vi "Velociprobe_Nanopositioner_Control_RT_2.vi"() -> ()   [LabVIEW 2015] (continued)
      tunnel: [w40 w68 w536 w697 w743 w798 w825 w917] -> w15
      tunnel: [w38 w67 w537 w696 w744 w796 w823 w915] -> w14
      tunnel: w13 -> [w37 w72 w540 w700 w747 w799 w828 w920]
      tunnel: w12 -> [_ w71 w541 w701 w748 w800 w829 w921]
      frame "Initialization", Default {
        w54 = 0  # IRQ Number(s)
        n8 = xnode "Open FPGA VI Reference"("error in"=w37) -> ("FPGA VI Reference Out"=w36:refnum<k20>, "error out"=w49:errorcluster)  [unwired: 1 in]
        n9 = xnode "Invoke Method"("FPGA VI Reference In"=w36, "error in"=w49, "Requested Depth"="Requested Depth") -> ("FPGA VI Reference Out"=w48:refnum<k20>, "error out"=w47:errorcluster, "Actual Depth"=→"Actual Depth":u32)
        n10 = xnode "Read/Write Control"("FPGA VI Reference In"=w48, "error in"=w47, "Datalog Time Period (uSec)"="Datalog Time Period (uSec)", "Datalog Cases"="Datalog Cases", "Interrupt Boolean"=FALSE) -> ("FPGA VI Reference Out"=w46:refnum<k20>, "error out"=w45:errorcluster)
        n11 = xnode "Invoke Method"("FPGA VI Reference In"=w46, "error in"=w45, "IRQ Number(s)"=w54, "Timeout (ms)"="IRQ Timeout (ms)") -> ("FPGA VI Reference Out"=w44:refnum<k20>, "error out"=w43:errorcluster, "Timed Out"=→"IRQ Timed Out":bool, "IRQ(s) Asserted"=w56:i32)
        n12 = xnode "Invoke Method"("FPGA VI Reference In"=w44, "error in"=w43, "IRQ Number(s)"=w56) -> ("FPGA VI Reference Out"=w42:refnum<k20>, "error out"=w41:errorcluster)
        n13 = disable-structure shown="Enabled" {
          disable-tunnel: [w64 errorcluster {"status"=FALSE, "code"=0, "source"=""} ("error out")] -> w50
          frame Disabled {
            n14 = invoke on="Waveform Graph 2" class="WFGraph (strict)" method="Reinit To Default"() -> (error out=w64:errorcluster)  [unwired: 3 in, 2 out]
          }
          frame Enabled {
          }
        }
        n15 = xnode "Read/Write Control"("FPGA VI Reference In"=w42, "error in"=w41) -> ("FPGA VI Reference Out"=w40:refnum<k20>, "error out"=w39:errorcluster, "error out (FPGA)"=w57:errorcluster)
        n16 = Merge Errors "Merge Errors"(w39, w57, w50) -> (w38:errorcluster)
        "Initialization error" <- w38
      }
      frame "Update Controller Info" {
        w296 = dbl[] [1.0, 2.0, 4.0, 5.0]  # Index_soscoeff_zz1
        w135 = dbl[] [1.0, 2.0, 4.0, 5.0]  # Index_soscoeff_yz1
        w156 = dbl[] [1.0, 2.0, 4.0, 5.0]  # Index_soscoeff_xz1
        w187 = dbl[] [1.0, 2.0, 4.0, 5.0]  # Index_soscoeff_zy1
        w317 = dbl[] [1.0, 2.0, 4.0, 5.0]  # Index_soscoeff_yy1
        w208 = dbl[] [1.0, 2.0, 4.0, 5.0]  # Index_soscoeff_xy1
        w234 = dbl[] [1.0, 2.0, 4.0, 5.0]  # Index_soscoeff_zx1
        w343 = dbl[] [1.0, 2.0, 4.0, 5.0]  # Index_soscoeff_xx1
        w260 = dbl[] [1.0, 2.0, 4.0, 5.0]  # Index_soscoeff_yx1
        w116 = "%.10f"  # format (%.3f)
        w124 = "%.10f"  # format (%.3f)
        w137 = "%.10f"  # format (%.3f)
        w145 = "%.10f"  # format (%.3f)
        w168 = "%.10f"  # format (%.3f)
        w176 = "%.10f"  # format (%.3f)
        w189 = "%.10f"  # format (%.3f)
        w197 = "%.10f"  # format (%.3f)
        w215 = "%.10f"  # format (%.3f)
        w223 = "%.10f"  # format (%.3f)
        w241 = "%.10f"  # format (%.3f)
        w249 = "%.10f"  # format (%.3f)
        w277 = "%.10f"  # format (%.3f)
        w285 = "%.10f"  # format (%.3f)
        w298 = "%.10f"  # format (%.3f)
        w306 = "%.10f"  # format (%.3f)
        w107 = fxp<+/-,42,9> 0.0 ("fixed-point type")
        w319 = "%.10f"  # format (%.3f)
        w106 = fxp<+/-,64,9> 0.0 ("fixed-point type")
        w332 = "%.10f"  # format (%.3f)
        w350 = 40000000.0  # FPGA Clock Rate (Hz)
        w83 = 1
        n17 = local read "sos gain SF Controller yy1c"() -> (w271:fxp<+/-,42,9>)
        n18 = local read "sos gain SF Controller yz1c"() -> (w92:fxp<+/-,42,9>)
        n19 = local read "sos gain SF Controller yx1c"() -> (w238:fxp<+/-,42,9>)
        n20 = local read "sos gain SF Controller xy1c"() -> (w161:fxp<+/-,42,9>)
        n21 = local read "sos gain SF Controller zy1c"() -> (w166:fxp<+/-,42,9>)
        n22 = local read "sos gain SF Controller xz1c"() -> (w108:fxp<+/-,42,9>)
        n23 = local read "sos gain SF Controller xx1c"() -> (w321:fxp<+/-,42,9>)
        n24 = local read "sos gain SF Controller zz1c"() -> (w269:fxp<+/-,42,9>)
        n25 = local read "sos gain SF Controller zx1c"() -> (w213:fxp<+/-,42,9>)
        n26 = local read "-a01(2) yy1c"() -> (w275:fxp<+/-,64,9>[])
        n27 = local read "-a02(2) yy1c"() -> (w274:fxp<+/-,64,9>[])
        n28 = local read "-a01(2) yz1c"() -> (w113:fxp<+/-,64,9>[])
        n29 = local read "-a02(2) yz1c"() -> (w114:fxp<+/-,64,9>[])
        n30 = local read "-a01(2) yx1c"() -> (w239:fxp<+/-,64,9>[])
        n31 = local read "-a02(2) yx1c"() -> (w235:fxp<+/-,64,9>[])
        n32 = local read "-a01(2) xy1c"() -> (w157:fxp<+/-,64,9>[])
        n33 = local read "-a02(2) xy1c"() -> (w158:fxp<+/-,64,9>[])
        n34 = local read "-a01(2) zy1c"() -> (w162:fxp<+/-,64,9>[])
        n35 = local read "-a02(2) zy1c"() -> (w163:fxp<+/-,64,9>[])
        n36 = local read "-a01(2) xz1c"() -> (w112:fxp<+/-,64,9>[])
        n37 = local read "-a02(2) xz1c"() -> (w111:fxp<+/-,64,9>[])
        n38 = local read "-a01(2) xx1c"() -> (w330:fxp<+/-,64,9>[])
        n39 = local read "-a02(2) xx1c"() -> (w329:fxp<+/-,64,9>[])
        n40 = local read "-a01(2) zz1c"() -> (w270:fxp<+/-,64,9>[])
        n41 = local read "-a02(2) zz1c"() -> (w266:fxp<+/-,64,9>[])
        n42 = local read "-a01(2) zx1c"() -> (w209:fxp<+/-,64,9>[])
        n43 = local read "-a02(2) zx1c"() -> (w210:fxp<+/-,64,9>[])
        n44 = local read "b01(2) yy1c"() -> (w273:fxp<+/-,64,9>[])
        n45 = local read "b02(2) yy1c"() -> (w272:fxp<+/-,64,9>[])
        n46 = local read "b01(2) yz1c"() -> (w78:fxp<+/-,64,9>[])
        n47 = local read "b02(2) yz1c"() -> (w77:fxp<+/-,64,9>[])
        n48 = local read "b01(2) yx1c"() -> (w236:fxp<+/-,64,9>[])
        n49 = local read "b02(2) yx1c"() -> (w237:fxp<+/-,64,9>[])
        n50 = local read "b01(2) xy1c"() -> (w159:fxp<+/-,64,9>[])
        n51 = local read "b02(2) xy1c"() -> (w160:fxp<+/-,64,9>[])
        n52 = local read "b01(2) zy1c"() -> (w164:fxp<+/-,64,9>[])
        n53 = local read "b02(2) zy1c"() -> (w165:fxp<+/-,64,9>[])
        n54 = local read "b01(2) xz1c"() -> (w110:fxp<+/-,64,9>[])
        n55 = local read "b02(2) xz1c"() -> (w109:fxp<+/-,64,9>[])
        n56 = local read "b01(2) xx1c"() -> (w328:fxp<+/-,64,9>[])
        n57 = local read "b02(2) xx1c"() -> (w327:fxp<+/-,64,9>[])
        n58 = local read "b01(2) zz1c"() -> (w267:fxp<+/-,64,9>[])
        n59 = local read "b02(2) zz1c"() -> (w268:fxp<+/-,64,9>[])
        n60 = local read "b01(2) zx1c"() -> (w211:fxp<+/-,64,9>[])
        n61 = local read "b02(2) zx1c"() -> (w212:fxp<+/-,64,9>[])
        n62 = Or(x="Optics Z Reset", y="Reset All") -> (x .or. y?=w105:bool)
        n63 = Or(x="Sample Z Reset", y="Reset All") -> (x .or. y?=w102:bool)
        n64 = Or(x="Optics X Reset", y="Reset All") -> (x .or. y?=w264:bool)
        n65 = Or(x="Optics Y Reset", y="Reset All") -> (x .or. y?=w262:bool)
        n66 = Or(x="Sample X Reset", y="Reset All") -> (x .or. y?=w104:bool)
        n67 = Or(x="Sample Y Reset", y="Reset All") -> (x .or. y?=w103:bool)
        n68 = call-poly <vilib>:"Read Delimited Spreadsheet.vi"("file path (dialog if empty)"="file path soscoeff_xx1", "format (%.3f)"=w332) -> ("all rows"=w331:dbl[][])  [unwired: 8 in, 5 out]
        n69 = call-poly <vilib>:"Read Delimited Spreadsheet.vi"("file path (dialog if empty)"="file path soscoeff_zy1", "format (%.3f)"=w176) -> ("all rows"=w175:dbl[][])  [unwired: 8 in, 5 out]
        n70 = call-poly <vilib>:"Read Delimited Spreadsheet.vi"("file path (dialog if empty)"="file path soscoeff_xy1", "format (%.3f)"=w197) -> ("all rows"=w196:dbl[][])  [unwired: 8 in, 5 out]
        n71 = call-poly <vilib>:"Read Delimited Spreadsheet.vi"("file path (dialog if empty)"="file path soscoeff_zx1", "format (%.3f)"=w223) -> ("all rows"=w222:dbl[][])  [unwired: 8 in, 5 out]
        n72 = call-poly <vilib>:"Read Delimited Spreadsheet.vi"("file path (dialog if empty)"="file path soscoeff_xz1", "format (%.3f)"=w145) -> ("all rows"=w144:dbl[][])  [unwired: 8 in, 5 out]
        n73 = call-poly <vilib>:"Read Delimited Spreadsheet.vi"("file path (dialog if empty)"="file path soscoeff_yx1", "format (%.3f)"=w249) -> ("all rows"=w248:dbl[][])  [unwired: 8 in, 5 out]
        n74 = call-poly <vilib>:"Read Delimited Spreadsheet.vi"("file path (dialog if empty)"="file path soscoeff_yy1", "format (%.3f)"=w306) -> ("all rows"=w305:dbl[][])  [unwired: 8 in, 5 out]
        n75 = call-poly <vilib>:"Read Delimited Spreadsheet.vi"("file path (dialog if empty)"="file path soscoeff_yz1", "format (%.3f)"=w124) -> ("all rows"=w123:dbl[][])  [unwired: 8 in, 5 out]
        n76 = call-poly <vilib>:"Read Delimited Spreadsheet.vi"("file path (dialog if empty)"="file path soscoeff_zz1", "format (%.3f)"=w285) -> ("all rows"=w284:dbl[][])  [unwired: 8 in, 5 out]
        n77 = Transpose 2D Array(2D array=w331) -> (transposed array=w342:dbl[][])
        n78 = Transpose 2D Array(2D array=w175) -> (transposed array=w186:dbl[][])
        n79 = Transpose 2D Array(2D array=w196) -> (transposed array=w207:dbl[][])
        n80 = Transpose 2D Array(2D array=w222) -> (transposed array=w233:dbl[][])
        n81 = Transpose 2D Array(2D array=w144) -> (transposed array=w155:dbl[][])
        n82 = Transpose 2D Array(2D array=w248) -> (transposed array=w259:dbl[][])
        n83 = Transpose 2D Array(2D array=w305) -> (transposed array=w316:dbl[][])
        n84 = Transpose 2D Array(2D array=w123) -> (transposed array=w134:dbl[][])
        n85 = Transpose 2D Array(2D array=w284) -> (transposed array=w295:dbl[][])
        n86 = call-poly <vilib>:"Read Delimited Spreadsheet.vi"("file path (dialog if empty)"="file path sos gain SF Controller_xx1", "format (%.3f)"=w319) -> ("all rows"=w318:dbl[][])  [unwired: 8 in, 5 out]
        n87 = call-poly <vilib>:"Read Delimited Spreadsheet.vi"("file path (dialog if empty)"="file path sos gain SF Controller_zy1", "format (%.3f)"=w168) -> ("all rows"=w167:dbl[][])  [unwired: 8 in, 5 out]
        n88 = call-poly <vilib>:"Read Delimited Spreadsheet.vi"("file path (dialog if empty)"="file path sos gain SF Controller_xy1", "format (%.3f)"=w189) -> ("all rows"=w188:dbl[][])  [unwired: 8 in, 5 out]
        n89 = call-poly <vilib>:"Read Delimited Spreadsheet.vi"("file path (dialog if empty)"="file path sos gain SF Controller_zx1", "format (%.3f)"=w215) -> ("all rows"=w214:dbl[][])  [unwired: 8 in, 5 out]
        n90 = call-poly <vilib>:"Read Delimited Spreadsheet.vi"("file path (dialog if empty)"="file path sos gain SF Controller_xz1", "format (%.3f)"=w137) -> ("all rows"=w136:dbl[][])  [unwired: 8 in, 5 out]
        n91 = call-poly <vilib>:"Read Delimited Spreadsheet.vi"("file path (dialog if empty)"="file path sos gain SF Controller_yx1", "format (%.3f)"=w241) -> ("all rows"=w240:dbl[][])  [unwired: 8 in, 5 out]
        n92 = call-poly <vilib>:"Read Delimited Spreadsheet.vi"("file path (dialog if empty)"="file path sos gain SF Controller_yy1", "format (%.3f)"=w298) -> ("all rows"=w297:dbl[][])  [unwired: 8 in, 5 out]
        n93 = call-poly <vilib>:"Read Delimited Spreadsheet.vi"("file path (dialog if empty)"="file path sos gain SF Controller_yz1", "format (%.3f)"=w116) -> ("all rows"=w115:dbl[][])  [unwired: 8 in, 5 out]
        n94 = call-poly <vilib>:"Read Delimited Spreadsheet.vi"("file path (dialog if empty)"="file path sos gain SF Controller_zz1", "format (%.3f)"=w277) -> ("all rows"=w276:dbl[][])  [unwired: 8 in, 5 out]
        n95 = xnode "Read/Write Control"("FPGA VI Reference In"=w71, "error in"=w72, "Controller Time Period (uSec)"="Controller Time Period (uSec)", "Controller Output Time Period (uSec)"="Controller Output Time Period (uSec)", "System Loop Type"="System Loop Type", "Controller Output Upper Limit"="Controller Output Upper Limit", "Controller Output Lower Limit"="Controller Output Lower Limit", "X-Stage nm to V Scaling"="X-Stage nm to V Scaling", "X-Stage Scaling Direction"="X-Stage Scaling Direction", "Y-Stage nm to V Scaling"="Y-Stage nm to V Scaling", "Z-Stage nm to V Scaling"="Z-Stage nm to V Scaling", "Plant Output Time Period (uSec)"="Plant Output Time Period (uSec)", "Reset Optics X"=w264, "Reset Optics Y"=w262, "Reset Optics Z"=w105, "Reset Sample X"=w104, "Reset Sample Y"=w103, "Reset Sample Z"=w102, "Optics X Stage Resolution (nm)"="Optics X Stage Resolution (nm)", "Optics Y Stage Resolution (nm)"="Optics Y Stage Resolution (nm)", "Optics Z Stage Resolution (nm)"="Optics Z Stage Resolution (nm)", "Sample X Stage Resolution (nm)"="Sample X Stage Resolution (nm)", "Sample Y Stage Resolution (nm)"="Sample Y Stage Resolution (nm)", "Sample Z Stage Resolution (nm)"="Sample Z Stage Resolution (nm)", "Scaling mV to V"="Scaling mV to V", "-a01(2) xx1"=w330, "-a02(2) xx1"=w329, "b01(2) xx1"=w328, "b02(2) xx1"=w327, "sos gain SF Controller xx1"=w321, "-a01(2) yy1"=w275, "-a02(2) yy1"=w274, "b01(2) yy1"=w273, "b02(2) yy1"=w272, "sos gain SF Controller yy1"=w271, "-a01(2) zz1"=w270, "-a02(2) zz1"=w266, "b01(2) zz1"=w267, "b02(2) zz1"=w268, "sos gain SF Controller zz1"=w269, "-a01(2) yx1"=w239, "-a02(2) yx1"=w235, "b01(2) yx1"=w236, "b02(2) yx1"=w237, "sos gain SF Controller yx1"=w238, "-a01(2) zx1"=w209, "-a02(2) zx1"=w210, "b01(2) zx1"=w211, "b02(2) zx1"=w212, "sos gain SF Controller zx1"=w213, "-a01(2) xy1"=w157, "-a02(2) xy1"=w158, "b01(2) xy1"=w159, "b02(2) xy1"=w160, "sos gain SF Controller xy1"=w161, "-a01(2) zy1"=w162, "-a02(2) zy1"=w163, "b01(2) zy1"=w164, "b02(2) zy1"=w165, "sos gain SF Controller zy1"=w166, "-a01(2) xz1"=w112, "-a02(2) xz1"=w111, "b01(2) xz1"=w110, "b02(2) xz1"=w109, "sos gain SF Controller xz1"=w108, "-a01(2) yz1"=w113, "-a02(2) yz1"=w114, "b01(2) yz1"=w78, "b02(2) yz1"=w77, "sos gain SF Controller yz1"=w92, "Analog Input Time Period (uSec)"="Analog Input Time Period (uSec)", "Optics and or Sample Stage"="Optics and or Sample Stage", "Y-Stage Scaling Direction"="Y-Stage Scaling Direction", "Z-Stage Scaling Direction"="Z-Stage Scaling Direction") -> ("FPGA VI Reference Out"=w70:refnum<k20>, "error out"=w69:errorcluster)
        n96 = for {
          tunnel: w343 -> [w519] mode=indexing
          tunnel: w342 -> [w518]
          tunnel: [w517] -> _ mode=indexing
          shift-right: [w517] -> w334
          shift-left: _ -> [w516]
          shift-left: _ -> [w515]
          shift-left: _ -> [w514]
          tunnel: [w516] -> w335
          tunnel: [w515] -> w336
          tunnel: [w514] -> w337
          n97 = Index Array "Index Array"(array=w518, index (row)=w519) -> (element=w517:dbl[])  [unwired: 1 in]
        }
        n98 = Index Array(array=w318, index (row)=0 ("index (row) 6")) -> (element=w326:dbl[])  [unwired: 1 in]
        n99 = for {
          tunnel: w187 -> [w417] mode=indexing
          tunnel: w186 -> [w416]
          tunnel: [w415] -> _ mode=indexing
          shift-right: [w415] -> w178
          shift-left: _ -> [w414]
          shift-left: _ -> [w413]
          shift-left: _ -> [w412]
          tunnel: [w414] -> w179
          tunnel: [w413] -> w180
          tunnel: [w412] -> w181
          n100 = Index Array "Index Array"(array=w416, index (row)=w417) -> (element=w415:dbl[])  [unwired: 1 in]
        }
        n101 = Index Array(array=w167, index (row)=0 ("index (row) 18")) -> (element=w174:dbl[])  [unwired: 1 in]
        n102 = for {
          tunnel: w208 -> [w434] mode=indexing
          tunnel: w207 -> [w433]
          tunnel: [w432] -> _ mode=indexing
          shift-right: [w432] -> w199
          shift-left: _ -> [w431]
          shift-left: _ -> [w430]
          shift-left: _ -> [w429]
          tunnel: [w431] -> w200
          tunnel: [w430] -> w201
          tunnel: [w429] -> w202
          n103 = Index Array "Index Array"(array=w433, index (row)=w434) -> (element=w432:dbl[])  [unwired: 1 in]
        }
        n104 = Index Array(array=w188, index (row)=0 ("index (row) 16")) -> (element=w195:dbl[])  [unwired: 1 in]
        n105 = for {
          tunnel: w234 -> [w451] mode=indexing
          tunnel: w233 -> [w450]
          tunnel: [w449] -> _ mode=indexing
          shift-right: [w449] -> w225
          shift-left: _ -> [w448]
          shift-left: _ -> [w447]
          shift-left: _ -> [w446]
          tunnel: [w448] -> w226
          tunnel: [w447] -> w227
          tunnel: [w446] -> w228
          n106 = Index Array "Index Array"(array=w450, index (row)=w451) -> (element=w449:dbl[])  [unwired: 1 in]
        }
        n107 = Index Array(array=w214, index (row)=0 ("index (row) 14")) -> (element=w221:dbl[])  [unwired: 1 in]
        n108 = for {
          tunnel: w156 -> [w400] mode=indexing
          tunnel: w155 -> [w399]
          tunnel: [w398] -> _ mode=indexing
          shift-right: [w398] -> w147
          shift-left: _ -> [w397]
          shift-left: _ -> [w396]
          shift-left: _ -> [w395]
          tunnel: [w397] -> w148
          tunnel: [w396] -> w149
          tunnel: [w395] -> w150
          n109 = Index Array "Index Array"(array=w399, index (row)=w400) -> (element=w398:dbl[])  [unwired: 1 in]
        }
        n110 = Index Array(array=w136, index (row)=0 ("index (row) 20")) -> (element=w143:dbl[])  [unwired: 1 in]
        n111 = for {
          tunnel: w260 -> [w468] mode=indexing
          tunnel: w259 -> [w467]
          tunnel: [w466] -> _ mode=indexing
          shift-right: [w466] -> w251
          shift-left: _ -> [w465]
          shift-left: _ -> [w464]
          shift-left: _ -> [w463]
          tunnel: [w465] -> w252
          tunnel: [w464] -> w253
          tunnel: [w463] -> w254
          n112 = Index Array "Index Array"(array=w467, index (row)=w468) -> (element=w466:dbl[])  [unwired: 1 in]
        }
        n113 = Index Array(array=w240, index (row)=0 ("index (row) 12")) -> (element=w247:dbl[])  [unwired: 1 in]
        n114 = for {
          tunnel: w317 -> [w502] mode=indexing
          tunnel: w316 -> [w501]
          tunnel: [w500] -> _ mode=indexing
          shift-right: [w500] -> w308
          shift-left: _ -> [w499]
          shift-left: _ -> [w498]
          shift-left: _ -> [w497]
          tunnel: [w499] -> w309
          tunnel: [w498] -> w310
          tunnel: [w497] -> w311
          n115 = Index Array "Index Array"(array=w501, index (row)=w502) -> (element=w500:dbl[])  [unwired: 1 in]
        }
        n116 = Index Array(array=w297, index (row)=0 ("index (row) 8")) -> (element=w304:dbl[])  [unwired: 1 in]
        n117 = for {
          tunnel: w135 -> [w383] mode=indexing
          tunnel: w134 -> [w382]
          tunnel: [w381] -> _ mode=indexing
          shift-right: [w381] -> w126
          shift-left: _ -> [w380]
          shift-left: _ -> [w379]
          shift-left: _ -> [w378]
          tunnel: [w380] -> w127
          tunnel: [w379] -> w128
          tunnel: [w378] -> w129
          n118 = Index Array "Index Array"(array=w382, index (row)=w383) -> (element=w381:dbl[])  [unwired: 1 in]
        }
        n119 = Index Array(array=w115, index (row)=0 ("index (row) 22")) -> (element=w122:dbl[])  [unwired: 1 in]
        n120 = Index Array(array=w276, index (row)=0 ("index (row) 10")) -> (element=w283:dbl[])  [unwired: 1 in]
        n121 = for {
          tunnel: w296 -> [w485] mode=indexing
          tunnel: w295 -> [w484]
          tunnel: [w483] -> _ mode=indexing
          shift-right: [w483] -> w287
          shift-left: _ -> [w482]
          shift-left: _ -> [w481]
          shift-left: _ -> [w480]
          tunnel: [w482] -> w288
          tunnel: [w481] -> w289
          tunnel: [w480] -> w290
          n122 = Index Array "Index Array"(array=w484, index (row)=w485) -> (element=w483:dbl[])  [unwired: 1 in]
        }
        n123 = Index Array(array=w326, index=0 ("index (row) 7")) -> (element=w324:dbl)
        n124 = Index Array(array=w174, index=0 ("index (row) 19")) -> (element=w172:dbl)
        n125 = Index Array(array=w195, index=0 ("index (row) 17")) -> (element=w193:dbl)
        n126 = Index Array(array=w221, index=0 ("index (row) 15")) -> (element=w219:dbl)
        n127 = Index Array(array=w143, index=0 ("index (row) 21")) -> (element=w141:dbl)
        n128 = Index Array(array=w247, index=0 ("index (row) 13")) -> (element=w245:dbl)
        n129 = Index Array(array=w304, index=0 ("index (row) 9")) -> (element=w302:dbl)
        n130 = Index Array(array=w122, index=0 ("index (row) 23")) -> (element=w120:dbl)
        n131 = Index Array(array=w283, index=0 ("index (row) 11")) -> (element=w281:dbl)
        n132 = xnode "Read/Write Control"("FPGA VI Reference In"=w70, "error in"=w69) -> ("FPGA VI Reference Out"=w68:refnum<k20>, "error out"=w67:errorcluster, "PI X-Stage Input (V)"=→"PI X-Stage Input (V)":fxp<+/-,20,5>, "PI Y-Stage Input (V)"=→"PI Y-Stage Input (V)":fxp<+/-,20,5>, "PI Z-Stage Input (V)"=→"PI Z-Stage Input (V)":fxp<+/-,20,5>, "X-Stage Input In Range?"=→"X-Stage Input In Range?":bool, "Y-Stage Input In Range?"=→"Y-Stage Input In Range?":bool, "Z-Stage Input In Range?"=→"Z-Stage Input In Range?":bool, "Measured Controller Time Period (Ticks)"=w351:u32, "Measured Controller Output Time Period (Ticks)"=w348:u32, "Measured Plant Output Time Period (Ticks)"=w84:u32, "Measured Analog Input Time Period (Ticks)"=→"Measured Analog Input Time Period (Ticks)":u32)
        "Measured Controller Time Period (Ticks)" <- w351
        "Measured Controller Output Time Period (Ticks)" <- w348
        "Measured Plant Output Time Period (Ticks)" <- w84
        n133 = To Fixed-Point(fixed-point type=w107, number=w193) -> (fixed-point=→"sos gain SF Controller xy1c":fxp<+/-,42,9>)
        n134 = To Fixed-Point(fixed-point type=w107, number=w302) -> (fixed-point=→"sos gain SF Controller yy1c":fxp<+/-,42,9>)
        n135 = To Fixed-Point(fixed-point type=w107, number=w172) -> (fixed-point=→"sos gain SF Controller zy1c":fxp<+/-,42,9>)
        n136 = To Fixed-Point(fixed-point type=w107, number=w141) -> (fixed-point=→"sos gain SF Controller xz1c":fxp<+/-,42,9>)
        n137 = To Fixed-Point(fixed-point type=w107, number=w120) -> (fixed-point=→"sos gain SF Controller yz1c":fxp<+/-,42,9>)
        n138 = To Fixed-Point(fixed-point type=w107, number=w245) -> (fixed-point=→"sos gain SF Controller yx1c":fxp<+/-,42,9>)
        n139 = To Fixed-Point(fixed-point type=w107, number=w219) -> (fixed-point=→"sos gain SF Controller zx1c":fxp<+/-,42,9>)
        n140 = To Fixed-Point(fixed-point type=w107, number=w281) -> (fixed-point=→"sos gain SF Controller zz1c":fxp<+/-,42,9>)
        n141 = To Fixed-Point(fixed-point type=w107, number=w324) -> (fixed-point=→"sos gain SF Controller xx1c":fxp<+/-,42,9>)
        n142 = Divide(x=w83, y=w350) -> (x/y=w85:dbl)
        n143 = Multiply(x=w85, y=w351) -> (x*y=w352:dbl)
        "Measured Controller Loop Rate (secs)" <- w352
        n144 = Multiply(x=w85, y=w348) -> (x*y=w360:dbl)
        "Measured Controller Output Loop Rate (secs)" <- w360
        n145 = Multiply(x=w85, y=w84) -> (x*y=w356:dbl)
        "Measured Plant Output Loop Rate (secs)" <- w356
        n146 = Multiply(x=w85, y=w84) -> (x*y=w89:dbl)
        "Measured Analog Input Loop Rate (secs)" <- w89
        n147 = for {
          tunnel: w179 -> [w428] mode=indexing
          tunnel: [w427] -> w185 mode=indexing
          tunnel: w178 -> [w426] mode=indexing
          tunnel: w181 -> [w425] mode=indexing
          tunnel: w180 -> [w424] mode=indexing
          tunnel: [w423] -> w184 mode=indexing
          tunnel: [w422] -> w183 mode=indexing
          tunnel: [w421] -> w182 mode=indexing
          tunnel: w106 -> [w418]
          n148 = Negate(x=w428) -> (-x=w420:dbl)
          n149 = Negate(x=w426) -> (-x=w419:dbl)
          n150 = To Fixed-Point(fixed-point type=w418, number=w420) -> (fixed-point=w427:fxp<+/-,64,9>)
          n151 = To Fixed-Point(fixed-point type=w418, number=w419) -> (fixed-point=w423:fxp<+/-,64,9>)
          n152 = To Fixed-Point(fixed-point type=w418, number=w425) -> (fixed-point=w422:fxp<+/-,64,9>)
          n153 = To Fixed-Point(fixed-point type=w418, number=w424) -> (fixed-point=w421:fxp<+/-,64,9>)
        }
        "-a01(2) zy1c" <- w185
        "-a02(2) zy1c" <- w184
        "b01(2) zy1c" <- w183
        "b02(2) zy1c" <- w182
        n154 = for {
          tunnel: w335 -> [w530] mode=indexing
          tunnel: [w529] -> w341 mode=indexing
          tunnel: w334 -> [w528] mode=indexing
          tunnel: w337 -> [w527] mode=indexing
          tunnel: w336 -> [w526] mode=indexing
          tunnel: [w525] -> w340 mode=indexing
          tunnel: [w524] -> w339 mode=indexing
          tunnel: [w523] -> w338 mode=indexing
          tunnel: w106 -> [w520]
          n155 = Negate(x=w530) -> (-x=w522:dbl)
          n156 = Negate(x=w528) -> (-x=w521:dbl)
          n157 = To Fixed-Point(fixed-point type=w520, number=w522) -> (fixed-point=w529:fxp<+/-,64,9>)
          n158 = To Fixed-Point(fixed-point type=w520, number=w521) -> (fixed-point=w525:fxp<+/-,64,9>)
          n159 = To Fixed-Point(fixed-point type=w520, number=w527) -> (fixed-point=w524:fxp<+/-,64,9>)
          n160 = To Fixed-Point(fixed-point type=w520, number=w526) -> (fixed-point=w523:fxp<+/-,64,9>)
        }
        "-a01(2) xx1c" <- w341
        "-a02(2) xx1c" <- w340
        "b01(2) xx1c" <- w339
        "b02(2) xx1c" <- w338
        n161 = for {
          tunnel: w200 -> [w445] mode=indexing
          tunnel: [w444] -> w206 mode=indexing
          tunnel: w199 -> [w443] mode=indexing
          tunnel: w202 -> [w442] mode=indexing
          tunnel: w201 -> [w441] mode=indexing
          tunnel: [w440] -> w205 mode=indexing
          tunnel: [w439] -> w204 mode=indexing
          tunnel: [w438] -> w203 mode=indexing
          tunnel: w106 -> [w435]
          n162 = Negate(x=w445) -> (-x=w437:dbl)
          n163 = Negate(x=w443) -> (-x=w436:dbl)
          n164 = To Fixed-Point(fixed-point type=w435, number=w437) -> (fixed-point=w444:fxp<+/-,64,9>)
          n165 = To Fixed-Point(fixed-point type=w435, number=w436) -> (fixed-point=w440:fxp<+/-,64,9>)
          n166 = To Fixed-Point(fixed-point type=w435, number=w442) -> (fixed-point=w439:fxp<+/-,64,9>)
          n167 = To Fixed-Point(fixed-point type=w435, number=w441) -> (fixed-point=w438:fxp<+/-,64,9>)
        }
        "-a01(2) xy1c" <- w206
        "-a02(2) xy1c" <- w205
        "b01(2) xy1c" <- w204
        "b02(2) xy1c" <- w203
        n168 = for {
          tunnel: w148 -> [w411] mode=indexing
          tunnel: [w410] -> w154 mode=indexing
          tunnel: w147 -> [w409] mode=indexing
          tunnel: w150 -> [w408] mode=indexing
          tunnel: w149 -> [w407] mode=indexing
          tunnel: [w406] -> w153 mode=indexing
          tunnel: [w405] -> w152 mode=indexing
          tunnel: [w404] -> w151 mode=indexing
          tunnel: w106 -> [w401]
          n169 = Negate(x=w411) -> (-x=w403:dbl)
          n170 = Negate(x=w409) -> (-x=w402:dbl)
          n171 = To Fixed-Point(fixed-point type=w401, number=w403) -> (fixed-point=w410:fxp<+/-,64,9>)
          n172 = To Fixed-Point(fixed-point type=w401, number=w402) -> (fixed-point=w406:fxp<+/-,64,9>)
          n173 = To Fixed-Point(fixed-point type=w401, number=w408) -> (fixed-point=w405:fxp<+/-,64,9>)
          n174 = To Fixed-Point(fixed-point type=w401, number=w407) -> (fixed-point=w404:fxp<+/-,64,9>)
        }
        "-a01(2) xz1c" <- w154
        "-a02(2) xz1c" <- w153
        "b01(2) xz1c" <- w152
        "b02(2) xz1c" <- w151
        n175 = for {
          tunnel: w309 -> [w513] mode=indexing
          tunnel: [w512] -> w315 mode=indexing
          tunnel: w308 -> [w511] mode=indexing
          tunnel: w311 -> [w510] mode=indexing
          tunnel: w310 -> [w509] mode=indexing
          tunnel: [w508] -> w314 mode=indexing
          tunnel: [w507] -> w313 mode=indexing
          tunnel: [w506] -> w312 mode=indexing
          tunnel: w106 -> [w503]
          n176 = Negate(x=w513) -> (-x=w505:dbl)
          n177 = Negate(x=w511) -> (-x=w504:dbl)
          n178 = To Fixed-Point(fixed-point type=w503, number=w505) -> (fixed-point=w512:fxp<+/-,64,9>)
          n179 = To Fixed-Point(fixed-point type=w503, number=w504) -> (fixed-point=w508:fxp<+/-,64,9>)
          n180 = To Fixed-Point(fixed-point type=w503, number=w510) -> (fixed-point=w507:fxp<+/-,64,9>)
          n181 = To Fixed-Point(fixed-point type=w503, number=w509) -> (fixed-point=w506:fxp<+/-,64,9>)
        }
        "-a01(2) yy1c" <- w315
        "-a02(2) yy1c" <- w314
        "b01(2) yy1c" <- w313
        "b02(2) yy1c" <- w312
        n182 = for {
          tunnel: w226 -> [w462] mode=indexing
          tunnel: [w461] -> w232 mode=indexing
          tunnel: w225 -> [w460] mode=indexing
          tunnel: w228 -> [w459] mode=indexing
          tunnel: w227 -> [w458] mode=indexing
          tunnel: [w457] -> w231 mode=indexing
          tunnel: [w456] -> w230 mode=indexing
          tunnel: [w455] -> w229 mode=indexing
          tunnel: w106 -> [w452]
          n183 = Negate(x=w462) -> (-x=w454:dbl)
          n184 = Negate(x=w460) -> (-x=w453:dbl)
          n185 = To Fixed-Point(fixed-point type=w452, number=w454) -> (fixed-point=w461:fxp<+/-,64,9>)
          n186 = To Fixed-Point(fixed-point type=w452, number=w453) -> (fixed-point=w457:fxp<+/-,64,9>)
          n187 = To Fixed-Point(fixed-point type=w452, number=w459) -> (fixed-point=w456:fxp<+/-,64,9>)
          n188 = To Fixed-Point(fixed-point type=w452, number=w458) -> (fixed-point=w455:fxp<+/-,64,9>)
        }
        "-a01(2) zx1c" <- w232
        "-a02(2) zx1c" <- w231
        "b01(2) zx1c" <- w230
        "b02(2) zx1c" <- w229
        n189 = for {
          tunnel: w252 -> [w479] mode=indexing
          tunnel: [w478] -> w258 mode=indexing
          tunnel: w251 -> [w477] mode=indexing
          tunnel: w254 -> [w476] mode=indexing
          tunnel: w253 -> [w475] mode=indexing
          tunnel: [w474] -> w257 mode=indexing
          tunnel: [w473] -> w256 mode=indexing
          tunnel: [w472] -> w255 mode=indexing
          tunnel: w106 -> [w469]
          n190 = Negate(x=w479) -> (-x=w471:dbl)
          n191 = Negate(x=w477) -> (-x=w470:dbl)
          n192 = To Fixed-Point(fixed-point type=w469, number=w471) -> (fixed-point=w478:fxp<+/-,64,9>)
          n193 = To Fixed-Point(fixed-point type=w469, number=w470) -> (fixed-point=w474:fxp<+/-,64,9>)
          n194 = To Fixed-Point(fixed-point type=w469, number=w476) -> (fixed-point=w473:fxp<+/-,64,9>)
          n195 = To Fixed-Point(fixed-point type=w469, number=w475) -> (fixed-point=w472:fxp<+/-,64,9>)
        }
        "-a01(2) yx1c" <- w258
        "-a02(2) yx1c" <- w257
        "b01(2) yx1c" <- w256
        "b02(2) yx1c" <- w255
        n196 = for {
          tunnel: w127 -> [w394] mode=indexing
          tunnel: [w393] -> w133 mode=indexing
          tunnel: w126 -> [w392] mode=indexing
          tunnel: w129 -> [w391] mode=indexing
          tunnel: w128 -> [w390] mode=indexing
          tunnel: [w389] -> w132 mode=indexing
          tunnel: [w388] -> w131 mode=indexing
          tunnel: [w387] -> w130 mode=indexing
          tunnel: w106 -> [w384]
          n197 = Negate(x=w394) -> (-x=w386:dbl)
          n198 = Negate(x=w392) -> (-x=w385:dbl)
          n199 = To Fixed-Point(fixed-point type=w384, number=w386) -> (fixed-point=w393:fxp<+/-,64,9>)
          n200 = To Fixed-Point(fixed-point type=w384, number=w385) -> (fixed-point=w389:fxp<+/-,64,9>)
          n201 = To Fixed-Point(fixed-point type=w384, number=w391) -> (fixed-point=w388:fxp<+/-,64,9>)
          n202 = To Fixed-Point(fixed-point type=w384, number=w390) -> (fixed-point=w387:fxp<+/-,64,9>)
        }
        "-a01(2) yz1c" <- w133
        "-a02(2) yz1c" <- w132
        "b01(2) yz1c" <- w131
        "b02(2) yz1c" <- w130
        n203 = Divide(x=w83, y=w352) -> (x/y=w363:dbl)
        n204 = Divide(x=w83, y=w360) -> (x/y=w359:dbl)
        n205 = Divide(x=w83, y=w356) -> (x/y=w355:dbl)
        n206 = for {
          tunnel: w288 -> [w496] mode=indexing
          tunnel: [w495] -> w294 mode=indexing
          tunnel: w287 -> [w494] mode=indexing
          tunnel: w290 -> [w493] mode=indexing
          tunnel: w289 -> [w492] mode=indexing
          tunnel: [w491] -> w293 mode=indexing
          tunnel: [w490] -> w292 mode=indexing
          tunnel: [w489] -> w291 mode=indexing
          tunnel: w106 -> [w486]
          n207 = Negate(x=w496) -> (-x=w488:dbl)
          n208 = Negate(x=w494) -> (-x=w487:dbl)
          n209 = To Fixed-Point(fixed-point type=w486, number=w488) -> (fixed-point=w495:fxp<+/-,64,9>)
          n210 = To Fixed-Point(fixed-point type=w486, number=w487) -> (fixed-point=w491:fxp<+/-,64,9>)
          n211 = To Fixed-Point(fixed-point type=w486, number=w493) -> (fixed-point=w490:fxp<+/-,64,9>)
          n212 = To Fixed-Point(fixed-point type=w486, number=w492) -> (fixed-point=w489:fxp<+/-,64,9>)
        }
        "-a01(2) zz1c" <- w294
        "-a02(2) zz1c" <- w293
        "b01(2) zz1c" <- w292
        "b02(2) zz1c" <- w291
        n213 = Divide(x=w83, y=w89) -> (x/y=w88:dbl)
        n214 = Divide(x=w363, y=1000) -> (x/y=→"Measured Controller Loop Rate (kHz)":dbl)
        n215 = Divide(x=w359, y=1000) -> (x/y=→"Measured Controller Output Loop Rate (kHz)":dbl)
        n216 = Divide(x=w355, y=1000) -> (x/y=→"Measured Plant Output Loop Rate (kHz)":dbl)
        n217 = Divide(x=w88, y=1000) -> (x/y=→"Measured Analog Input Loop Rate (kHz)":dbl)
      }
      frame "Update Reference Info" {
        w608 = 40000000.0  # FPGA Clock Rate (Hz)
        w602 = 1
        w615 = 40000000.0  # FPGA Clock Rate (Hz)
        w609 = 1
        w620 = errorcluster {"status"=FALSE, "code"=0, "source"=""}  # error in (no error)
        w623 = errorcluster {"status"=FALSE, "code"=0, "source"=""}  # error in (no error)
        w637 = 40000000.0  # FPGA Clock Rate (Hz)
        w631 = 1
        w649 = errorcluster {"status"=FALSE, "code"=0, "source"=""}  # error in (no error)
        w616 = 40000000.0  # FPGA clock rate (Hz)
        n218 = case shown="\"EPICS Snake Scan\"" "Snake Scan Reference FPGA or EPICS" {
          tunnel: ["X Ramp Start (nm)" w667] -> w549
          tunnel: ["X Ramp End (nm)" w666] -> w548
          tunnel: ["Fly Scan Start" w672] -> w547
          tunnel: ["Y Ramp Start (nm)" w665] -> w546
          tunnel: ["Y Ramp End (nm)" w664] -> w545
          tunnel: ["Y Step Size (nm)" w668] -> w544
          tunnel: ["X Step Size (nm)" w671] -> w543
          tunnel: [w658 w669] -> w542
          tunnel: ["Y Step Size (nm)" w668] -> w535
          tunnel: ["X Ramp Start (nm)" w667] -> w534
          tunnel: ["X Ramp End (nm)" w666] -> w533
          tunnel: ["Y Ramp Start (nm)" w665] -> w532
          tunnel: ["Y Ramp End (nm)" w664] -> w531
          frame "FPGA Snake Scan", Default {
            n219 = local read "DT Frequency (Hz)"() -> (w658:dbl)
          }
          frame "EPICS Snake Scan" {
            w670 = fxp<+/-,16,16> 0.0 ("fixed-point type")
            n220 = shared-variable "RT CompactRIO Target\\RT_EPICS_Shared_Variables.lvlib\\2iddVELO:VP:Trigger_Freq_Hz"() -> (w669:dbl)  [unwired: 1 in, 1 out]
            "2iddVELO:VP:Trigger_Freq_Hz" <- w669
            n221 = shared-variable "RT CompactRIO Target\\RT_EPICS_Shared_Variables.lvlib\\2iddVELO:VP:Y_Step_Size_nm"() -> (w674:dbl)  [unwired: 1 in, 1 out]
            "2iddVELO:VP:Y_Step_Size_nm" <- w674
            n222 = shared-variable "RT CompactRIO Target\\RT_EPICS_Shared_Variables.lvlib\\2iddVELO:VP:X_Step_Size_nm"() -> (w673:dbl)  [unwired: 1 in, 1 out]
            "2iddVELO:VP:X_Step_Size_nm" <- w673
            n223 = shared-variable "RT CompactRIO Target\\RT_EPICS_Shared_Variables.lvlib\\2iddVELO:VP:Y_Start_nm"() -> (w675:dbl)  [unwired: 1 in, 1 out]
            n224 = shared-variable "RT CompactRIO Target\\RT_EPICS_Shared_Variables.lvlib\\2iddVELO:VP:Y_End_nm"() -> (w663:dbl)  [unwired: 1 in, 1 out]
            n225 = shared-variable "RT CompactRIO Target\\RT_EPICS_Shared_Variables.lvlib\\2iddVELO:VP:Flyscan_Start"() -> (w672:bool)  [unwired: 1 in, 1 out]
            "2iddVELO:VP:Flyscan_Start" <- w672
            n226 = shared-variable "RT CompactRIO Target\\RT_EPICS_Shared_Variables.lvlib\\2iddVELO:VP:X_Start_nm"() -> (w677:dbl)  [unwired: 1 in, 1 out]
            "2iddVELO:VP:X_Start_nm" <- w677
            n227 = shared-variable "RT CompactRIO Target\\RT_EPICS_Shared_Variables.lvlib\\2iddVELO:VP:X_End_nm"() -> (w676:dbl)  [unwired: 1 in, 1 out]
            "2iddVELO:VP:X_End_nm" <- w676
            n228 = Negate(x=w663) -> (-x=w662:dbl)
            "2iddVELO:VP:Y_End_nm" <- w662
            n229 = Negate(x=w675) -> (-x=w661:dbl)
            "2iddVELO:VP:Y_Start_nm" <- w661
            n230 = To Fixed-Point(fixed-point type=w670, number=w677) -> (fixed-point=w667:fxp<+/-,16,16>)
            n231 = To Fixed-Point(fixed-point type=w670, number=w676) -> (fixed-point=w666:fxp<+/-,16,16>)
            n232 = To Fixed-Point(fixed-point type=w670, number=w661) -> (fixed-point=w665:fxp<+/-,16,16>)
            n233 = To Fixed-Point(fixed-point type=w670, number=w662) -> (fixed-point=w664:fxp<+/-,16,16>)
            n234 = To Fixed-Point(fixed-point type=w670, number=w674) -> (fixed-point=w668:fxp<+/-,16,16>)
            n235 = To Fixed-Point(fixed-point type=w670, number=w673) -> (fixed-point=w671:fxp<+/-,16,16>)
          }
        }
        n236 = local read "X Ramp Period (usec)"() -> (w551:fxp<+,24,24>)
        n237 = local read "Y Ramp Period (usec)"() -> (w552:fxp<+,24,24>)
        n238 = case shown="\"Constant\", Default" "Z Reference Wave Selection" {
          tunnel: "Z frequency (Hz)" -> [w678 w679 w681 w683 w684]
          tunnel: [w678 w679 w680 w683 w684] -> w577
          tunnel: w576 -> [_ _ w682 _ _]
          frame "Constant", Default {
          }
          frame "Sine Wave" {
          }
          frame "Sawtooth Wave" {
            n239 = Multiply(x=w682, y=w681) -> (x*y=w680:dbl)
          }
          frame "Square Wave" {
          }
          frame "Filtered White Noise" {
          }
        }
        n240 = case shown="\"Constant\", Default" "Y Reference Wave Selection" {
          tunnel: "Y frequency (Hz)" -> [w685 w686 w687 w688]
          tunnel: [w685 w686 w687 w688] -> w582
          tunnel: w579 -> [_ _ _ _]
          frame "Constant", Default {
          }
          frame "Sine Wave" {
          }
          frame "Custom Ramp Wave" {
          }
          frame "Filtered White Noise" {
          }
        }
        n241 = case shown="\"Custom Up Down Ramp\"" "X Reference Wave Selection" {
          tunnel: "X frequency (Hz)" -> [w689 w690 w691 w692]
          tunnel: [w689 w690 w691 w692] -> w586
          tunnel: w584 -> [_ _ _ _]
          frame "Constant", Default {
          }
          frame "Sine Wave" {
          }
          frame "Custom Up Down Ramp" {
          }
          frame "Filtered White Noise" {
          }
        }
        n242 = call <vilib>:"Normalize Signal Generation Parameters.vi"("frequency (Hz)"=w582, "FPGA clock rate (Hz)"=w616, "phase offset (deg)"="Y phase offset (deg)", "error in (no error)"=w623) -> ("frequency (periods/tick)"=w619:fxp<+,32,0>, "phase offset (periods)"=w618:fxp<+,32,0>, "error out"=→"error out (Sig Gen) 2":errorcluster)  [unwired: 6 in, 3 out]
        "Y frequency (periods/tick)" <- w619
        "Y phase offset (periods)" <- w618
        n243 = call <vilib>:"Normalize Signal Generation Parameters.vi"("frequency (Hz)"=w577, "FPGA clock rate (Hz)"=w616, "phase offset (deg)"="Z phase offset (deg)", "error in (no error)"=w620) -> ("frequency (periods/tick)"=w617:fxp<+,32,0>, "phase offset (periods)"=w595:fxp<+,32,0>, "error out"=→"error out (Sig Gen) 3":errorcluster)  [unwired: 6 in, 3 out]
        "Z frequency (periods/tick)" <- w617
        "Z phase offset (periods)" <- w595
        n244 = call <vilib>:"Normalize Signal Generation Parameters.vi"("frequency (Hz)"=w586, "FPGA clock rate (Hz)"=w616, "phase offset (deg)"="X phase offset (deg)", "error in (no error)"=w649) -> ("frequency (periods/tick)"=w648:fxp<+,32,0>, "phase offset (periods)"=w626:fxp<+,32,0>, "error out"=→"error out (Sig Gen)":errorcluster)  [unwired: 6 in, 3 out]
        "X frequency (periods/tick)" <- w648
        "X phase offset (periods)" <- w626
        n245 = xnode "Read/Write Control"("FPGA VI Reference In"=w541, "error in"=w540, "X Reference Time Period (uSec)"="X Reference Time Period (uSec)", "Y Reference Time Period (uSec)"="Y Reference Time Period (uSec)", "Z Reference Time Period (uSec)"="Z Reference Time Period (uSec)", "X Reference Wave Selection"="X Reference Wave Selection", "Y Reference Wave Selection"="Y Reference Wave Selection", "Z Reference Wave Selection"="Z Reference Wave Selection", "X Reference Reset"="X Reference Reset", "Y Reference Reset"="Y Reference Reset", "Z Reference Reset"="Z Reference Reset", "X Reference Amplitude (nm)"="X Reference Amplitude (nm)", "Y Reference Amplitude (nm)"="Y Reference Amplitude (nm)", "Z Reference Amplitude (nm)"="Z Reference Amplitude (nm)", "X Frequency (periods/tick)"=w648, "X Phase Offset (periods)"=w626, "Y Frequency (periods/tick)"=w619, "Y Phase Offset (periods)"=w618, "Z Frequency (periods/tick)"=w617, "Z Phase Offset (periods)"=w595, "X Reference DC Offset (nm)"="X Reference DC Offset (nm)", "Y Reference DC Offset (nm)"="Y Reference DC Offset (nm)", "Z Reference DC Offset (nm)"="Z Reference DC Offset (nm)", "X White Noise Amplitude"="X White Noise Amplitude", "X White Noise Seed"="X White Noise Seed", "Y White Noise Amplitude"="Y White Noise Amplitude", "Y White Noise Seed"="Y White Noise Seed", "Z White Noise Amplitude"="Z White Noise Amplitude", "Z White Noise Seed"="Z White Noise Seed", "Mod 3 AI0 V to nm Scaling"="Mod 3 AI0 V to nm Scaling", "Mod 3 AI1 V to nm Scaling"="Mod 3 AI1 V to nm Scaling", "Mod 3 AI2 V to nm Scaling"="Mod 3 AI2 V to nm Scaling", "X Ramp Period (usec)"=w551, "X Ramp Start (nm)"=w549, "X Ramp End (nm)"=w548, "X Start Marker (nm)"="X Start Marker (nm)", "Fly Scan Start"=w547, "Y Ramp Period (usec)"=w552, "Y Ramp Start (nm)"=w546, "Y Ramp End (nm)"=w545, "Y Ramp Drop Size (nm)"=w544, "Y Start Marker (nm)"="Y Start Marker (nm)") -> ("FPGA VI Reference Out"=w539:refnum<k20>, "error out"=w538:errorcluster)